vi "Dresden R2R Sputter 03.02.2018 IY24.vi"() -> ()   [LabVIEW 2009] (continued)
                                frame #1 {
                                n19691 = local read "Semi"() -> (w24342:bool)
                                n19692 = case shown="False" w24342 {
                                frame #0 {
                                n19693 = local write "Ch3_PA7"(TRUE ("PA3")) -> ()
                                n19694 = Wait Until Next ms Multiple(millisecond multiple=u32 1000) -> ()  [unwired: 1 out]
                                }
                                frame #1 {
                                }
                                }
                                }
                                }
                              }
                              frame #1 {
                              }
                            }
                          }
                          frame #2 {
                            # "CLOSE BG-BV"
                            n19695 = local read "Semi"() -> (w24345:bool)
                            n19696 = case shown="False" w24345 {
                              frame #0 {
                                n19697 = stacked-sequence {
                                frame #0 {
                                n19698 = local read "Semi"() -> (w24346:bool)
                                n19699 = case shown="False" w24346 {
                                frame #0 {
                                n19700 = while {
                                i -> [w24353]
                                stop <- w24347 stop-if-true
                                n19701 = Greater?(x=w24353, y=50) -> (0:w24351:bool)
                                n19702 = case shown="True" w24351 {
                                frame #0 {
                                }
                                frame #1 {
                                n19703 = local write "Semi"(TRUE ("Semi")) -> ()
                                n19704 = local write "Error Message"("Start up process  cancelled\nbecause  BG-BV not closed.\nPlease check  BG-BV3 connections." ("Error Message")) -> ()
                                }
                                }
                                n19705 = local read "Ch3_Bg_bv_di"() -> (w24350:bool)
                                n19706 = case shown="True" w24350 {
                                tunnel: [TRUE FALSE] -> w24349
                                frame #0 {
                                }
                                frame #1 {
                                n19707 = Wait Until Next ms Multiple(millisecond multiple=u32 200) -> ()  [unwired: 1 out]
                                n19708 = local write "Ch3_Bg_bv_do"(FALSE ("Ch1_Tp_bv_do")) -> ()
                                }
                                }
                                n19709 = local read "Semi"() -> (w24348:bool)
                                n19710 = Or(x=w24349, y=w24348) -> (x .or. y?=w24347:bool)
                                }
                                }
                                frame #1 {
                                }
                                }
                                }
                                frame #1 {
                                n19711 = local read "Semi"() -> (w24360:bool)
                                n19712 = case shown="False" w24360 {
                                frame #0 {
                                n19713 = local write "Ch3_PA8"(TRUE ("PA3")) -> ()
                                n19714 = Wait Until Next ms Multiple(millisecond multiple=u32 1000) -> ()  [unwired: 1 out]
                                }
                                frame #1 {
                                }
                                }
                                }
                                }
                              }
                              frame #1 {
                              }
                            }
                          }
                          frame #3 {
                            # "CLOSE TP-BV"
                            n19715 = local read "Semi"() -> (w24363:bool)
                            n19716 = case shown="False" w24363 {
                              frame #0 {
                                n19717 = stacked-sequence {
                                frame #0 {
                                n19718 = local read "Semi"() -> (w24364:bool)
                                n19719 = case shown="False" w24364 {
                                frame #0 {
                                n19720 = while {
                                i -> [w24371]
                                stop <- w24365 stop-if-true
                                n19721 = Greater?(x=w24371, y=50) -> (0:w24369:bool)
                                n19722 = case shown="True" w24369 {
                                frame #0 {
                                }
                                frame #1 {
                                n19723 = local write "Semi"(TRUE ("Semi")) -> ()
                                n19724 = local write "Error Message"("Start up process  cancelled\nbecause  TP-BV not closed.\nPlease check  TP3-BV connections." ("Error Message")) -> ()
                                }
                                }
                                n19725 = local read "Ch3_Tp_bv_di"() -> (w24368:bool)
                                n19726 = case shown="True" w24368 {
                                tunnel: [TRUE FALSE] -> w24367
                                frame #0 {
                                }
                                frame #1 {
                                n19727 = Wait Until Next ms Multiple(millisecond multiple=u32 200) -> ()  [unwired: 1 out]
                                n19728 = local write "Ch3_Tp_bv_do"(FALSE ("Ch1_Tp_bv_do")) -> ()
                                }
                                }
                                n19729 = local read "Semi"() -> (w24366:bool)
                                n19730 = Or(x=w24367, y=w24366) -> (x .or. y?=w24365:bool)
                                }
                                }
                                frame #1 {
                                }
                                }
                                }
                                frame #1 {
                                n19731 = local read "Semi"() -> (w24378:bool)
                                n19732 = case shown="False" w24378 {
                                frame #0 {
                                n19733 = Wait Until Next ms Multiple(millisecond multiple=u32 1000) -> ()  [unwired: 1 out]
                                n19734 = local write "Ch3_PA9"(TRUE ("PA5")) -> ()
                                }
                                frame #1 {
                                }
                                }
                                }
                                }
                              }
                              frame #1 {
                              }
                            }
                          }
                          frame #4 {
                            # "False PL-ATM"
                            n19735 = local read "Semi"() -> (w24381:bool)
                            n19736 = case shown="False" w24381 {
                              frame #0 {
                                n19737 = stacked-sequence {
                                frame #0 {
                                n19738 = local read "Semi"() -> (w24382:bool)
                                n19739 = case shown="False" w24382 {
                                frame #0 {
                                n19740 = local write "Ch3_Pl_atm_do"(FALSE ("Ch1_Pl_atm_do")) -> ()
                                }
                                frame #1 {
                                }
                                }
                                }
                                frame #1 {
                                n19741 = local read "Semi"() -> (w24384:bool)
                                n19742 = case shown="False" w24384 {
                                frame #0 {
                                n19743 = local write "Ch3_PA10"(TRUE ("PA3")) -> ()
                                n19744 = Wait Until Next ms Multiple(millisecond multiple=u32 1000) -> ()  [unwired: 1 out]
                                }
                                frame #1 {
                                }
                                }
                                }
                                }
                              }
                              frame #1 {
                              }
                            }
                          }
                          frame #5 {
                            # "STOP MP"
                            n19745 = local read "Semi"() -> (w24387:bool)
                            n19746 = case shown="False" w24387 {
                              frame #0 {
                                n19747 = stacked-sequence {
                                frame #0 {
                                n19748 = local read "Semi"() -> (w24388:bool)
                                n19749 = case shown="False" w24388 {
                                frame #0 {
                                n19750 = while {
                                i -> [w24395]
                                stop <- w24389 stop-if-true
                                n19751 = Greater?(x=w24395, y=50) -> (0:w24393:bool)
                                n19752 = case shown="True" w24393 {
                                frame #0 {
                                }
                                frame #1 {
                                n19753 = local write "Semi"(TRUE ("Semi")) -> ()
                                n19754 = local write "Error Message"("Start up process  cancelled\nbecause MP not stopped.\nPlease check MP3 connections." ("Error Message")) -> ()
                                }
                                }
                                n19755 = local read "Ch3_Mp_di"() -> (w24392:bool)
                                n19756 = case shown="True" w24392 {
                                tunnel: [TRUE FALSE] -> w24391
                                frame #0 {
                                }
                                frame #1 {
                                n19757 = Wait Until Next ms Multiple(millisecond multiple=u32 200) -> ()  [unwired: 1 out]
                                n19758 = local write "Ch3_Mp_do"(FALSE ("Ch1_Tp_bv_do")) -> ()
                                }
                                }
                                n19759 = local read "Semi"() -> (w24390:bool)
                                n19760 = Or(x=w24391, y=w24390) -> (x .or. y?=w24389:bool)
                                }
                                }
                                frame #1 {
                                }
                                }
                                }
                                frame #1 {
                                n19761 = local read "Semi"() -> (w24402:bool)
                                n19762 = case shown="False" w24402 {
                                frame #0 {
                                n19763 = Wait Until Next ms Multiple(millisecond multiple=u32 1000) -> ()  [unwired: 1 out]
                                n19764 = local write "Ch3_PA11"(TRUE ("PA3")) -> ()
                                }
                                frame #1 {
                                }
                                }
                                }
                                }
                              }
                              frame #1 {
                              }
                            }
                          }
                          frame #6 {
                            # "OPEN PL-VBV"
                            n19765 = local read "Semi"() -> (w24405:bool)
                            n19766 = case shown="False" w24405 {
                              frame #0 {
                                n19767 = stacked-sequence {
                                frame #0 {
                                n19768 = local read "Semi"() -> (w24406:bool)
                                n19769 = case shown="False" w24406 {
                                frame #0 {
                                n19770 = while {
                                i -> [w24413]
                                stop <- w24408 stop-if-true
                                n19771 = Greater?(x=w24413, y=50) -> (0:w24411:bool)
                                n19772 = case shown="True" w24411 {
                                frame #0 {
                                }
                                frame #1 {
                                n19773 = local write "Semi"(TRUE ("Semi")) -> ()
                                n19774 = local write "Error Message"("Start up process  cancelled\nbecause  PL-VBV not opened.\nPlease check PL-VBV3 connections." ("Error Message")) -> ()
                                }
                                }
                                n19775 = local read "Ch3_Pl_atm_di"() -> (w24407:bool)
                                n19776 = case shown="False" w24407 {
                                tunnel: [w24415 TRUE] -> w24410
                                frame #0 {
                                n19777 = local read "Ch3_Pl_vbv_di"() -> (w24414:bool)
                                n19778 = case shown="False" w24414 {
                                tunnel: [FALSE TRUE] -> w24415
                                frame #0 {
                                n19779 = Wait Until Next ms Multiple(millisecond multiple=u32 200) -> ()  [unwired: 1 out]
                                n19780 = local write "Ch3_Pl_vbv_do"(TRUE ("Ch1_Tp_bv_do")) -> ()
                                }
                                frame #1 {
                                }
                                }
                                }
                                frame #1 {
                                }
                                }
                                n19781 = local read "Semi"() -> (w24409:bool)
                                n19782 = Or(x=w24410, y=w24409) -> (x .or. y?=w24408:bool)
                                }
                                }
                                frame #1 {
                                }
                                }
                                }
                                frame #1 {
                                n19783 = local read "Semi"() -> (w24423:bool)
                                n19784 = case shown="False" w24423 {
                                frame #0 {
                                n19785 = local write "Ch3_PA12"(TRUE ("PA3")) -> ()
                                n19786 = Wait Until Next ms Multiple(millisecond multiple=u32 1000) -> ()  [unwired: 1 out]
                                }
                                frame #1 {
                                }
                                }
                                }
                                }
                              }
                              frame #1 {
                              }
                            }
                          }
                          frame #7 {
                            # "CHECK PL-PRESSURE"
                            n19787 = local read "Semi"() -> (w24426:bool)
                            n19788 = case shown="False" w24426 {
                              frame #0 {
                                n19789 = stacked-sequence {
                                frame #0 {
                                n19790 = local read "Semi"() -> (w24427:bool)
                                n19791 = case shown="False" w24427 {
                                frame #0 {
                                n19792 = while {
                                i -> [w24434]
                                stop <- w24429 stop-if-true
                                n19793 = Greater?(x=w24434, y=50) -> (0:w24432:bool)
                                n19794 = case shown="True" w24432 {
                                frame #0 {
                                }
                                frame #1 {
                                n19795 = local write "Semi"(TRUE ("Semi")) -> ()
                                n19796 = local write "Error Message"("Start up process  cancelled\nbecause  PL-ATM not opened.\nPlease check PL-ATM3 connections." ("Error Message")) -> ()
                                }
                                }
                                n19797 = local read "Ch3_Pl_atm_di"() -> (w24428:bool)
                                n19798 = case shown="True" w24428 {
                                tunnel: [FALSE TRUE] -> w24431
                                frame #0 {
                                }
                                frame #1 {
                                n19799 = Wait Until Next ms Multiple(millisecond multiple=u32 500) -> ()  [unwired: 1 out]
                                }
                                }
                                n19800 = local read "Semi"() -> (w24430:bool)
                                n19801 = Or(x=w24431, y=w24430) -> (x .or. y?=w24429:bool)
                                }
                                }
                                frame #1 {
                                }
                                }
                                }
                                frame #1 {
                                n19802 = local read "Semi"() -> (w24440:bool)
                                n19803 = case shown="False" w24440 {
                                frame #0 {
                                n19804 = local write "Ch3_PA13"(TRUE ("PA3")) -> ()
                                n19805 = Wait Until Next ms Multiple(millisecond multiple=u32 1000) -> ()  [unwired: 1 out]
                                }
                                frame #1 {
                                }
                                }
                                }
                                }
                              }
                              frame #1 {
                              }
                            }
                          }
                          frame #8 {
                            # "False CH-ATM"
                            n19806 = local read "Semi"() -> (w24443:bool)
                            n19807 = case shown="False" w24443 {
                              frame #0 {
                                n19808 = stacked-sequence {
                                frame #0 {
                                n19809 = local read "Semi"() -> (w24444:bool)
                                n19810 = case shown="False" w24444 {
                                frame #0 {
                                n19811 = local write "Ch3_Ch_atm_do"(FALSE ("Ch1_Pl_atm_do")) -> ()
                                }
                                frame #1 {
                                }
                                }
                                }
                                frame #1 {
                                n19812 = local read "Semi"() -> (w24446:bool)
                                n19813 = case shown="False" w24446 {
                                frame #0 {
                                n19814 = local write "Ch3_PA14"(TRUE ("PA3")) -> ()
                                n19815 = Wait Until Next ms Multiple(millisecond multiple=u32 1000) -> ()  [unwired: 1 out]
                                }
                                frame #1 {
                                }
                                }
                                }
                                }
                              }
                              frame #1 {
                              }
                            }
                          }
                          frame #9 {
                            # "OPEN PC-BV"
                            n19816 = local read "Semi"() -> (w24449:bool)
                            n19817 = case shown="False" w24449 {
                              frame #0 {
                                n19818 = stacked-sequence {
                                frame #0 {
                                n19819 = local read "Semi"() -> (w24450:bool)
                                n19820 = case shown="False" w24450 {
                                frame #0 {
                                n19821 = stacked-sequence {
                                frame #0 {
                                n19822 = local read "Semi"() -> (w24451:bool)
                                n19823 = case shown="False" w24451 {
                                frame #0 {
                                n19824 = local write "Pc_bv3_auto_open"(TRUE ("Tp1_auto_start")) -> ()
                                }
                                frame #1 {
                                }
                                }
                                }
                                frame #1 {
                                n19825 = local read "Semi"() -> (w24453:bool)
                                n19826 = case shown="False" w24453 {
                                frame #0 {
                                n19827 = Wait (ms)(milliseconds to wait=u32 1000) -> ()  [unwired: 1 out]
                                }
                                frame #1 {
                                }
                                }
                                }
                                frame #2 {
                                n19828 = local read "Semi"() -> (w24455:bool)
                                n19829 = case shown="False" w24455 {
                                frame #0 {
                                n19830 = while {
                                i -> [w24461]
                                stop <- w24457 stop-if-true
                                n19831 = local read "Pc_bv_opened_ch3"() -> (w24459:bool)
                                n19832 = Greater?(x=w24461, y=120) -> (0:w24460:bool)
                                n19833 = local read "Semi"() -> (w24458:bool)
                                n19834 = Compound Arithmetic op=OR(w24458, w24459, w24460) -> (w24457:bool)
                                n19835 = Wait (ms)(milliseconds to wait=u32 500) -> ()  [unwired: 1 out]
                                }
                                }
                                frame #1 {
                                }
                                }
                                }
                                frame #3 {
                                n19836 = local read "Semi"() -> (w24463:bool)
                                n19837 = case shown="False" w24463 {
                                frame #0 {
                                n19838 = local read "Pc_bv_opened_ch3"() -> (w24464:bool)
                                n19839 = case shown="False" w24464 {
                                frame #0 {
                                n19840 = local write "Pc_bv3_auto_open"(TRUE ("Pc_bv1_auto_open")) -> ()
                                }
                                frame #1 {
                                }
                                }
                                }
                                frame #1 {
                                }
                                }
                                }
                                frame #4 {
                                n19841 = local read "Semi"() -> (w24466:bool)
                                n19842 = case shown="False" w24466 {
                                frame #0 {
                                n19843 = local read "Pc_bv_opened_ch3"() -> (w24467:bool)
                                n19844 = case shown="False" w24467 {
                                frame #0 {
                                n19845 = Wait (ms)(milliseconds to wait=u32 1000) -> ()  [unwired: 1 out]
                                }
                                frame #1 {
                                }
                                }
                                }
                                frame #1 {
                                }
                                }
                                }
                                frame #5 {
                                n19846 = local read "Semi"() -> (w24469:bool)
                                n19847 = case shown="False" w24469 {
                                frame #0 {
                                n19848 = while {
                                i -> [w24475]
                                stop <- w24471 stop-if-true
                                n19849 = local read "Pc_bv_opened_ch3"() -> (w24473:bool)
                                n19850 = Greater?(x=w24475, y=120) -> (0:w24474:bool)
                                n19851 = local read "Semi"() -> (w24472:bool)
                                n19852 = Compound Arithmetic op=OR(w24472, w24473, w24474) -> (w24471:bool)
                                n19853 = Wait (ms)(milliseconds to wait=u32 500) -> ()  [unwired: 1 out]
                                }
                                }
                                frame #1 {
                                }
                                }
                                }
                                frame #6 {
                                n19854 = local read "Semi"() -> (w24477:bool)
                                n19855 = case shown="False" w24477 {
                                frame #0 {
                                n19856 = local read "Pc_bv_opened_ch3"() -> (w24478:bool)
                                n19857 = case shown="False" w24478 {
                                frame #0 {
                                n19858 = local write "Error Message"("Start up process  cancelled\nbecause  PC-BV not opened.\nPlease check PC-BV3 connections." ("Error Message")) -> ()
                                n19859 = Wait (ms)(milliseconds to wait=u32 1000) -> ()  [unwired: 1 out]
                                }
                                frame #1 {
                                }
                                }
                                }
                                frame #1 {
                                }
                                }
                                }
                                }
                                }
                                frame #1 {
                                }
                                }
                                }
                                frame #1 {
                                n19860 = local read "Semi"() -> (w24481:bool)
                                n19861 = case shown="False" w24481 {
                                frame #0 {
                                n19862 = local write "Ch3_PA15"(TRUE ("PA3")) -> ()
                                n19863 = Wait Until Next ms Multiple(millisecond multiple=u32 1000) -> ()  [unwired: 1 out]
                                }
                                frame #1 {
                                }
                                }
                                }
                                }
                              }
                              frame #1 {
                              }
                            }
                          }
                          frame #10 {
                            # "OPEN CH-VBV"
                            n19864 = local read "Semi"() -> (w24484:bool)
                            n19865 = case shown="False" w24484 {
                              frame #0 {
                                n19866 = stacked-sequence {
                                frame #0 {
                                n19867 = local read "Semi"() -> (w24485:bool)
                                n19868 = case shown="False" w24485 {
                                frame #0 {
                                n19869 = while {
                                i -> [w24492]
                                stop <- w24487 stop-if-true
                                n19870 = Greater?(x=w24492, y=50) -> (0:w24490:bool)
                                n19871 = case shown="True" w24490 {
                                frame #0 {
                                }
                                frame #1 {
                                n19872 = local write "Semi"(TRUE ("Semi")) -> ()
                                n19873 = local write "Error Message"("Start up process  cancelled\nbecause  CH-VBV not opened.\nPlease check  CH3-VBV connections." ("Error Message")) -> ()
                                }
                                }
                                n19874 = local read "Ch3_Ch_atm_di"() -> (w24486:bool)
                                n19875 = case shown="False" w24486 {
                                tunnel: [w24493 TRUE] -> w24489
                                frame #0 {
                                n19876 = local read "Ch3_Ch_vbv_di"() -> (w24494:bool)
                                n19877 = case shown="False" w24494 {
                                tunnel: [FALSE TRUE] -> w24493
                                frame #0 {
                                n19878 = local write "Ch3_Ch_vbv_do"(TRUE ("Ch1_Tp_bv_do")) -> ()
                                n19879 = Wait Until Next ms Multiple(millisecond multiple=u32 200) -> ()  [unwired: 1 out]
                                }
                                frame #1 {
                                }
                                }
                                }
                                frame #1 {
                                }
                                }
                                n19880 = local read "Semi"() -> (w24488:bool)
                                n19881 = Or(x=w24489, y=w24488) -> (x .or. y?=w24487:bool)
                                }
                                }
                                frame #1 {
                                }
                                }
                                }
                                frame #1 {
                                n19882 = local read "Semi"() -> (w24502:bool)
                                n19883 = case shown="False" w24502 {
                                frame #0 {
                                n19884 = local write "Ch3_PA16"(TRUE ("PA3")) -> ()
                                n19885 = Wait Until Next ms Multiple(millisecond multiple=u32 1000) -> ()  [unwired: 1 out]
                                }
                                frame #1 {
                                }
                                }
                                }
                                }
                              }
                              frame #1 {
                              }
                            }
                          }
                          frame #11 {
                            # "OPEN/CLOSE TRNS GV-BP2"
                            n19886 = local read "Semi"() -> (w24505:bool)
                            n19887 = case shown="False" w24505 {
                              frame #0 {
                                n19888 = stacked-sequence {
                                frame #0 {
                                n19889 = local read "Semi"() -> (w24506:bool)
                                n19890 = case shown="False" w24506 {
                                frame #0 {
                                n19891 = while {
                                i -> [w24515]
                                stop <- w24510 stop-if-true
                                n19892 = Greater?(x=w24515, y=800) -> (0:w24513:bool)
                                n19893 = case shown="True" w24513 {
                                frame #0 {
                                }
                                frame #1 {
                                n19894 = local read "Ch4pressure"() -> (w24535:dbl)
                                n19895 = Less?(x=w24535, y=1) -> (x < y?=w24534:bool)
                                n19896 = case shown="False" w24534 {
                                frame #0 {
                                n19897 = local write "Error Message"("Start up process  cancelled\nbecause \n Trns GV-BP2 not closed.\nPlease check \nTrns GV-BP2 connections." ("Error Message")) -> ()
                                }
                                frame #1 {
                                n19898 = local write "Error Message"("Start up process  cancelled\nbecause \n Trns GV-BP2 not opened.\nPlease check \nTrns GV-BP2 connections." ("Error Message")) -> ()
                                }
                                }
                                n19899 = local write "Semi"(TRUE ("Semi")) -> ()
                                }
                                }
                                n19900 = local read "Ch4pressure"() -> (w24509:dbl)
                                n19901 = Less?(x=w24509, y=1) -> (x < y?=w24507:bool)
                                n19902 = case shown="False" w24507 {
                                tunnel: [w24517 w24525] -> w24512
                                frame #0 {
                                n19903 = local read "Ch3_Trns_gv_bp2_di"() -> (w24516:bool)
                                n19904 = case shown="True" w24516 {
                                tunnel: [TRUE FALSE] -> w24517
                                frame #0 {
                                }
                                frame #1 {
                                n19905 = local write "Ch3_Trns_gv_bp2_do"(FALSE ("Ch1_Tp_bv_do")) -> ()
                                n19906 = Wait Until Next ms Multiple(millisecond multiple=u32 200) -> ()  [unwired: 1 out]
                                }
                                }
                                }
                                frame #1 {
                                n19907 = local read "Ch3_pressure"() -> (w24524:dbl)
                                n19908 = Greater Or Equal?(x=w24524, y=700.0) -> (x >= y?=w24522:bool)
                                n19909 = case shown="True" w24522 {
                                tunnel: [FALSE w24529] -> w24525
                                frame #0 {
                                n19910 = Wait Until Next ms Multiple(millisecond multiple=u32 500) -> ()  [unwired: 1 out]
                                }
                                frame #1 {
                                n19911 = local read "Ch3_Trns_gv_bp2_di"() -> (w24528:bool)
                                n19912 = case shown="False" w24528 {
                                tunnel: [FALSE TRUE] -> w24529
                                frame #0 {
                                n19913 = local write "Ch3_Trns_gv_bp2_do"(TRUE ("Ch1_Tp_bv_do")) -> ()
                                n19914 = Wait Until Next ms Multiple(millisecond multiple=u32 200) -> ()  [unwired: 1 out]
                                }
                                frame #1 {
                                }
                                }
                                }
                                }
                                }
                                }
                                n19915 = local read "Semi"() -> (w24511:bool)
                                n19916 = Or(x=w24512, y=w24511) -> (x .or. y?=w24510:bool)
                                }
                                }
                                frame #1 {
                                }
                                }
                                }
                                frame #1 {
                                n19917 = local read "Semi"() -> (w24540:bool)
                                n19918 = case shown="False" w24540 {
                                frame #0 {
                                n19919 = local write "Ch3_PA17"(TRUE ("PA3")) -> ()
                                n19920 = Wait Until Next ms Multiple(millisecond multiple=u32 1000) -> ()  [unwired: 1 out]
                                }
                                frame #1 {
                                }
                                }
                                }
                                }
                              }
                              frame #1 {
                              }
                            }
                          }
                          frame #12 {
                            # "OPEN/CLOSE TRNS GV-BP"
                            n19921 = local read "Semi"() -> (w24543:bool)
                            n19922 = case shown="False" w24543 {
                              frame #0 {
                                n19923 = stacked-sequence {
                                frame #0 {
                                n19924 = local read "Semi"() -> (w24544:bool)
                                n19925 = case shown="False" w24544 {
                                frame #0 {
                                n19926 = while {
                                i -> [w24553]
                                stop <- w24548 stop-if-true
                                n19927 = Greater?(x=w24553, y=800) -> (0:w24551:bool)
                                n19928 = case shown="True" w24551 {
                                frame #0 {
                                }
                                frame #1 {
                                n19929 = local read "Ch2_pressure"() -> (w24573:dbl)
                                n19930 = Less?(x=w24573, y=1) -> (x < y?=w24572:bool)
                                n19931 = case shown="True" w24572 {
                                frame #0 {
                                n19932 = local write "Error Message"("Start up process  cancelled\nbecause \n Trns GV-BP not closed.\nPlease check \nTrns GV-BP connections." ("Error Message")) -> ()
                                }
                                frame #1 {
                                n19933 = local write "Error Message"("Start up process  cancelled\nbecause\n  Trns GV-BP not opened.\nPlease check \nTrns GV-BP connections." ("Error Message")) -> ()
                                }
                                }
                                n19934 = local write "Semi"(TRUE ("Semi")) -> ()
                                }
                                }
                                n19935 = local read "Ch2_pressure"() -> (w24547:dbl)
                                n19936 = Less?(x=w24547, y=1) -> (x < y?=w24545:bool)
                                n19937 = case shown="True" w24545 {
                                tunnel: [w24555 w24563] -> w24550
                                frame #0 {
                                n19938 = local read "Ch3_Trns_gv_bp_di"() -> (w24554:bool)
                                n19939 = case shown="True" w24554 {
                                tunnel: [TRUE FALSE] -> w24555
                                frame #0 {
                                }
                                frame #1 {
                                n19940 = local write "Ch3_Trns_gv_bp_do"(FALSE ("Ch1_Tp_bv_do")) -> ()
                                n19941 = Wait Until Next ms Multiple(millisecond multiple=u32 200) -> ()  [unwired: 1 out]
                                }
                                }
                                }
                                frame #1 {
                                n19942 = local read "Ch3_pressure"() -> (w24562:dbl)
                                n19943 = Greater Or Equal?(x=w24562, y=700.0) -> (x >= y?=w24560:bool)
                                n19944 = case shown="True" w24560 {
                                tunnel: [FALSE w24567] -> w24563
                                frame #0 {
                                n19945 = Wait Until Next ms Multiple(millisecond multiple=u32 500) -> ()  [unwired: 1 out]
                                }
                                frame #1 {
                                n19946 = local read "Ch3_Trns_gv_bp_di"() -> (w24566:bool)
                                n19947 = case shown="False" w24566 {
                                tunnel: [FALSE TRUE] -> w24567
                                frame #0 {
                                n19948 = local write "Ch3_Trns_gv_bp_do"(TRUE ("Ch1_Tp_bv_do")) -> ()
                                n19949 = Wait Until Next ms Multiple(millisecond multiple=u32 200) -> ()  [unwired: 1 out]
                                }
                                frame #1 {
                                }
                                }
                                }
                                }
                                }
                                }
                                n19950 = local read "Semi"() -> (w24549:bool)
                                n19951 = Or(x=w24550, y=w24549) -> (x .or. y?=w24548:bool)
                                }
                                }
                                frame #1 {
                                }
                                }
                                }
                                frame #1 {
                                n19952 = local read "Semi"() -> (w24578:bool)
                                n19953 = case shown="False" w24578 {
                                frame #0 {
                                n19954 = local write "Ch3_PA18"(TRUE ("PA3")) -> ()
                                n19955 = Wait Until Next ms Multiple(millisecond multiple=u32 1000) -> ()  [unwired: 1 out]
                                }
                                frame #1 {
                                }
                                }
                                }
                                }
                              }
                              frame #1 {
                              }
                            }
                          }
                          frame #13 {
                            # "CHECK CH-ATM"
                            n19956 = local read "Semi"() -> (w24581:bool)
                            n19957 = case shown="False" w24581 {
                              frame #0 {
                                n19958 = stacked-sequence {
                                frame #0 {
                                n19959 = local read "Semi"() -> (w24582:bool)
                                n19960 = case shown="False" w24582 {
                                frame #0 {
                                n19961 = while {
                                i -> [w24589]
                                stop <- w24584 stop-if-true
                                n19962 = Greater?(x=w24589, y=1500) -> (0:w24587:bool)
                                n19963 = case shown="True" w24587 {
                                frame #0 {
                                }
                                frame #1 {
                                n19964 = local write "Semi"(TRUE ("Semi")) -> ()
                                n19965 = local write "Error Message"("Start up process  cancelled\nbecause  CH-ATM not opened.\nPlease check CH-ATM connections." ("Error Message")) -> ()
                                }
                                }
                                n19966 = local read "Ch3_Ch_atm_di"() -> (w24583:bool)
                                n19967 = case shown="False" w24583 {
                                tunnel: [FALSE TRUE] -> w24586
                                frame #0 {
                                n19968 = Wait Until Next ms Multiple(millisecond multiple=u32 500) -> ()  [unwired: 1 out]
                                }
                                frame #1 {
                                }
                                }
                                n19969 = local read "Semi"() -> (w24585:bool)
                                n19970 = Or(x=w24586, y=w24585) -> (x .or. y?=w24584:bool)
                                }
                                }
                                frame #1 {
                                }
                                }
                                }
                                frame #1 {
                                n19971 = local read "Semi"() -> (w24595:bool)
                                n19972 = case shown="False" w24595 {
                                frame #0 {
                                n19973 = local write "Ch3_PA19"(TRUE ("PA3")) -> ()
                                n19974 = Wait Until Next ms Multiple(millisecond multiple=u32 1000) -> ()  [unwired: 1 out]